vi "GrabFromBasler.vi"() -> ()   [LabVIEW 2012]
doc: "The Grab VI acquires images continuously and displays the images in an image control using high-level acquisition VIs. A grab is appropriate for high-speed applications in which you need to process only one image at a time."
uses:
  <vilib>/userdefined/High Color/IMAQdx.ctl
  <vilib>/vision/Image Controls.llb/IMAQ Image.ctl
panel:
  out "resulting string":string
  out "# of Particles found":i32
  in  "threshold":cluster{"Lower value":sgl, "Upper value":sgl}={"Lower value"=0.0, "Upper value"=100.0}
  in  "remove particle size":i32=5
  in  "Operation":u16(ring)=3 items=["AutoM", "Close", "Dilate", "Erode", "Gradient", "Gradient out", "Gradient in", "Hit miss", "Open", "PClose", "POpen", "Thick", "Thin"]
  in  "Interpolation Type 2":u32(ring)=1 items=["Zero Order", "Bi-Linear", "Quadratic", "Cubic Spline"]
  in  "downsampling 2":u32=10
  in  "exposure time (us)":u32=50000
  out "threholded":T1(plugin-control)
  out "single channel":T1(plugin-control)
  out "Image":T1(plugin-control)
  in  "stop":bool
  in  "height":u32=600
  in  "width":u32=2500
  in  "Camera Name":T2="cam0"
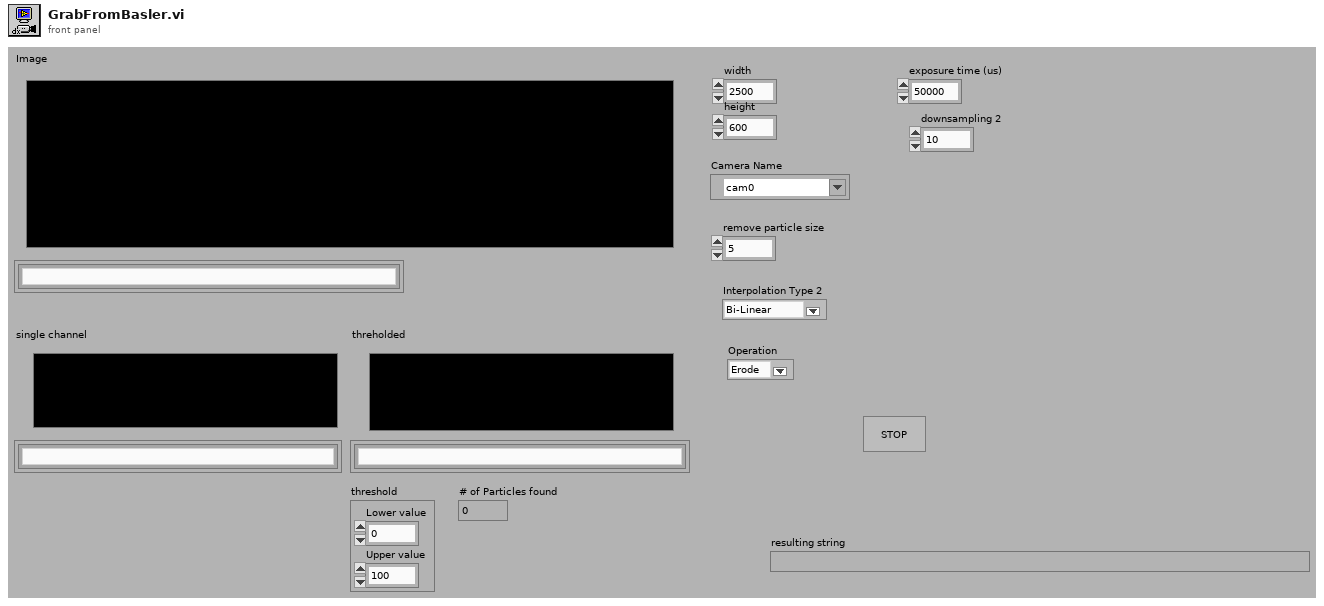
[diagram p1: front panel]
types:
  T1 = typedef "IMAQ Image.ctl" = refnum<image>
  T2 = typedef "IMAQdx.ctl" = refnum<k21>
  T3 = cluster{"Channel":i32, "Range":cluster{"Lower value":sgl, "Upper value":sgl}, "downsampling":u32, "Operation":u16, "Interpolation Type":u32, "remove particle size":i32, "Single channel":T1, "Thresholded":T1, "raw image":T1, "subimage":T1}
  T4 = cluster{"Buffer Number":u32, "Frame Rate":dbl, "# of Particles found":i32, "Image":T1, "Single channel":T1, "thresholded":T1, "status":bool}
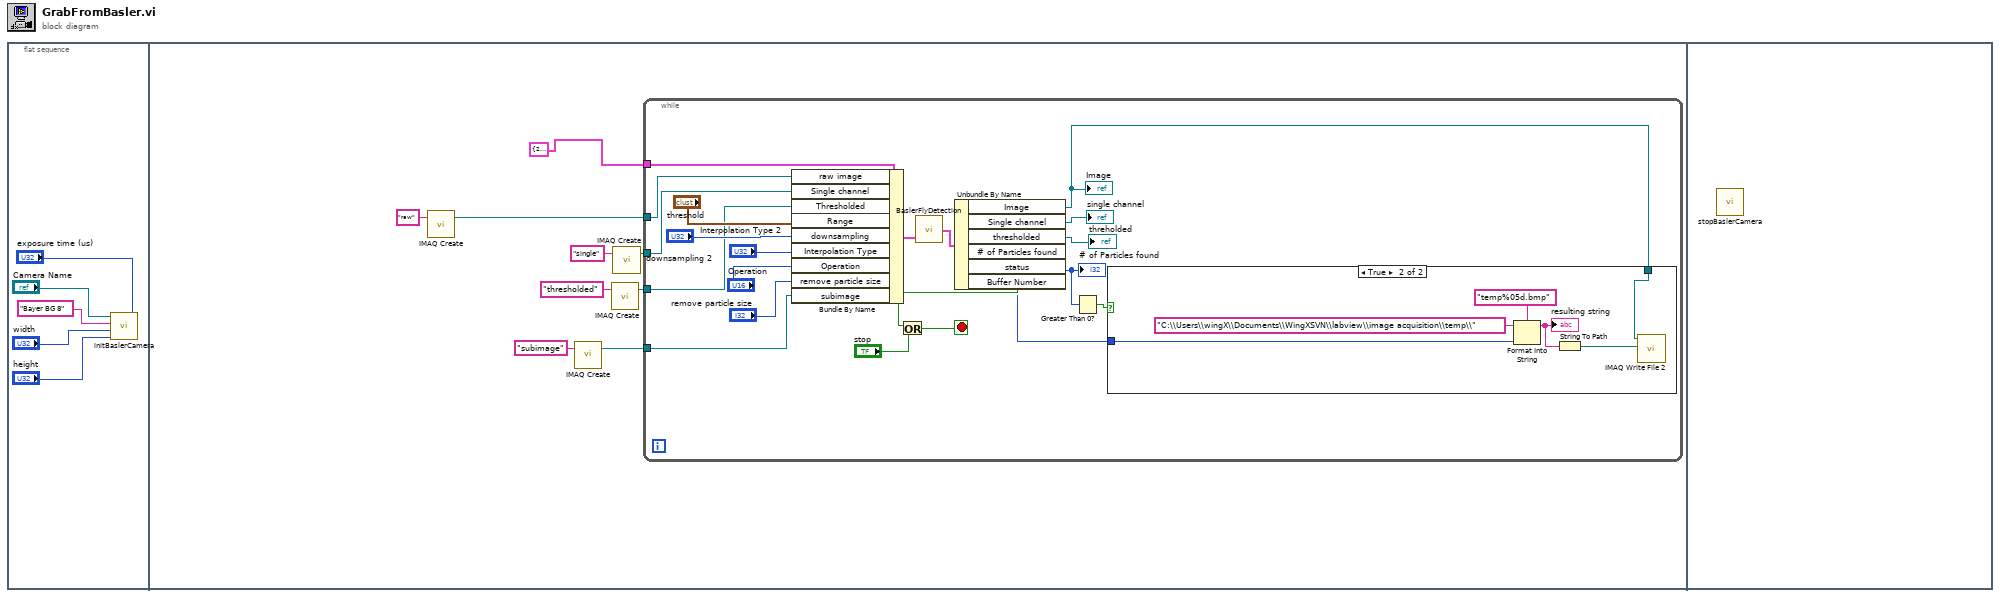
[diagram p0: block diagram]
diagram:
  n1 = flat-sequence {
    frame #0 {
      n2 = call "initBaslerCamera.vi"("exposure time (us)"="exposure time (us)", "height"="height", "width"="width", "Pixel Format"="Bayer BG 8" ("ValueString"), "Camera Name"="Camera Name") -> ()  [unwired: 2 in]
    }
    frame #1 {
      n3 = call "IMAQ Create"("Image Name"="raw") -> ("New Image"=w9:T1)  [unwired: 3 in, 2 out]
      n4 = call "IMAQ Create"("Image Name"="subimage") -> ("New Image"=w6:T1)  [unwired: 3 in, 2 out]
      n5 = call "IMAQ Create"("Image Name"="thresholded") -> ("New Image"=w13:T1)  [unwired: 3 in, 2 out]
      n6 = call "IMAQ Create"("Image Name"="single") -> ("New Image"=w14:T1)  [unwired: 3 in, 2 out]
      n7 = while {
        tunnel: w9 -> [w27]
        tunnel: w13 -> [w25]
        tunnel: w14 -> [w26]
        tunnel: T3 {"Channel"=2, "Range"={"Lower value"=0.0, "Upper value"=100.0}, "downsampling"=16, "Operation"=0, "Interpolation Type"=0, "remove particle size"=5, "Single channel"="single", "Thresholded"="thresholded", "raw image"="raw", "subimage"="subimage"} ("image processing controls") -> [w28]
        tunnel: w6 -> [w15]
        stop <- w34 stop-if-true
        n8 = Bundle By Name(cluster=w28, "raw image"=w27, "Single channel"=w26, "Thresholded"=w25, "Range"="threshold", "downsampling"="downsampling 2", "Interpolation Type"="Interpolation Type 2", "Operation"="Operation", "remove particle size"="remove particle size", "subimage"=w15) -> (w24:T3)
        n9 = call "BaslerFlyDetection.vi"("image processing controls"=w24) -> ("image processing indicators"=w23:T4)
        n10 = Unbundle By Name(w23) -> ("Image"=w16:T1, "Single channel"=→"single channel":T1, "thresholded"=→"threholded":T1, "# of Particles found"=w18:i32, "status"=w20:bool, "Buffer Number"=w17:u32)
        "Image" <- w16
        "# of Particles found" <- w18
        n11 = Or(x=w20, y="stop") -> (x .or. y?=w34:bool)
        n12 = Greater Than 0?(x=w18) -> (x > 0?=w19:bool)
        n13 = case shown="True" w19 {
          tunnel: w17 -> [_ w39]
          tunnel: w16 -> [_ w36]
          frame False {
          }
          frame True {
            n14 = Format Into String(format string="temp%05d.bmp", initial string="C:\\Users\\wingX\\Documents\\WingXSVN\\labview\\image acquisition\\temp\\", w39) -> (resulting string=w38:string)  [unwired: 1 in, 1 out]
            "resulting string" <- w38
            n15 = String To Path(string=w38) -> (path=w37:path)
            n16 = call-poly "IMAQ Write File 2"("File Path"=w37, "Image"=w36) -> ()  [unwired: 8 in, 2 out]
          }
        }
      }
    }
    frame #2 {
      n17 = call "stopBaslerCamera.vi"() -> ()  [unwired: 12 in]
    }
  }
